vi "_testStepCfgEditor.vi"() -> ()   [LabVIEW 2010]
panel:
  in  "Generate testStepCfg.ini":bool
  out "View row details":string[](array[string])
  in  "Library function":string(tree)="library function"
  in  "Test Step CFG EDIT":string[][](table)
  out "error out":errorcluster
  in  "error in":errorcluster
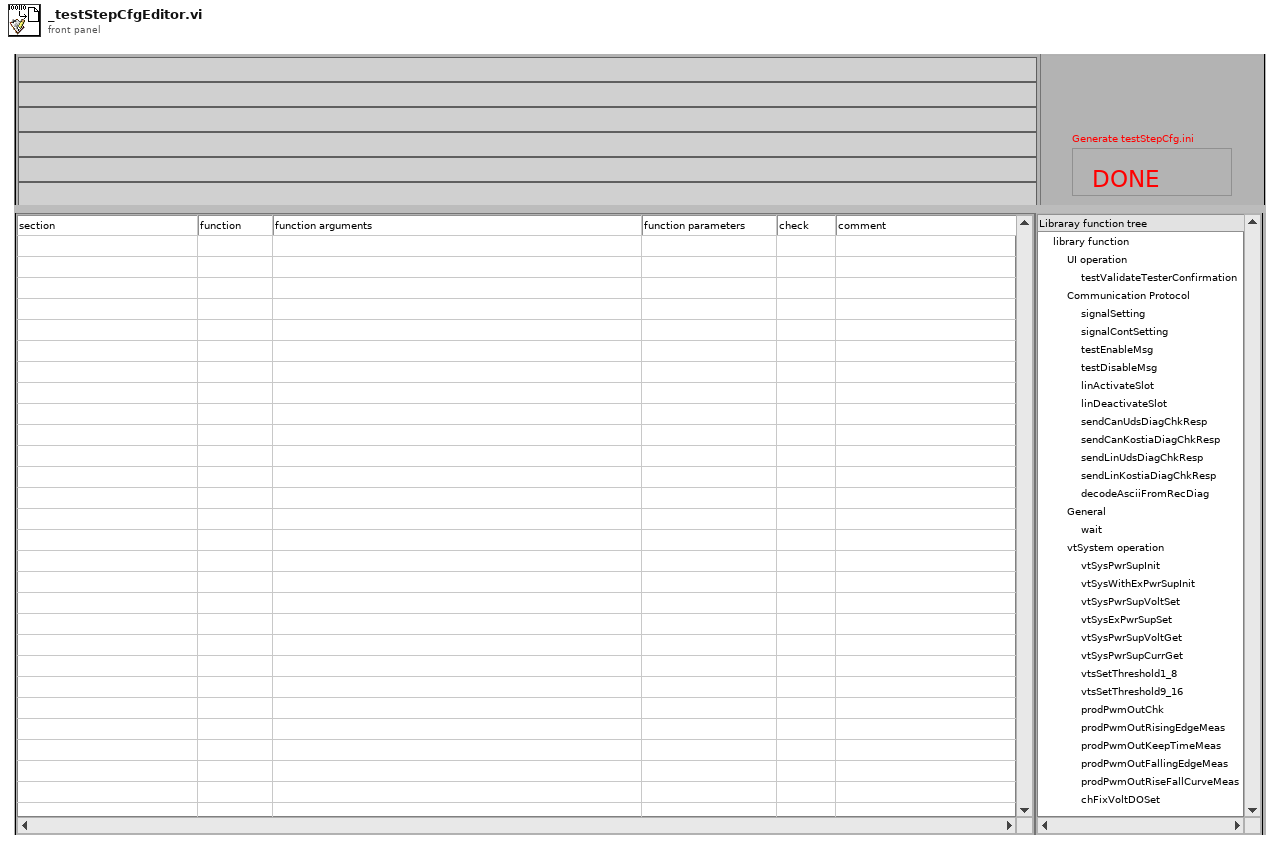
[diagram p1: front panel]
types:
  T1 = typedef "LVRowAndColumnTypeDef.ctl" = cluster{"Row":i32, "Column":i32}
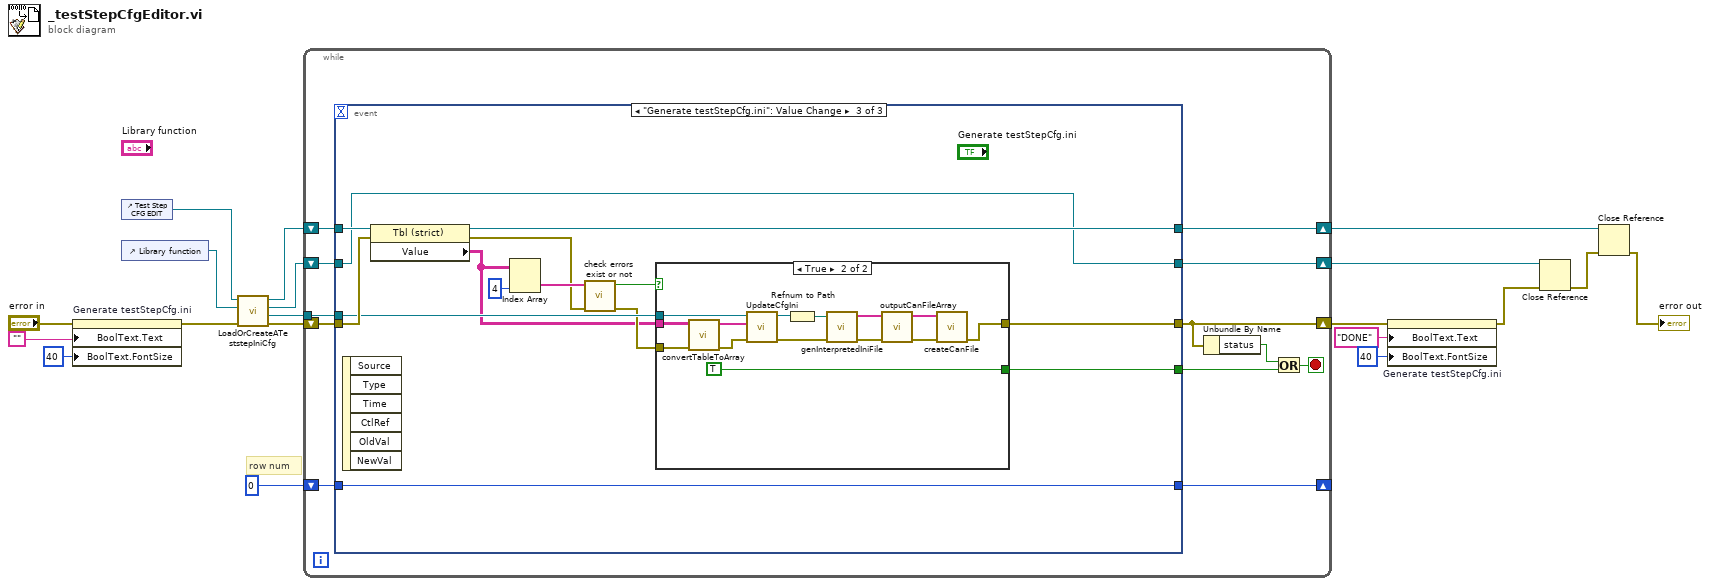
[diagram p0: block diagram]
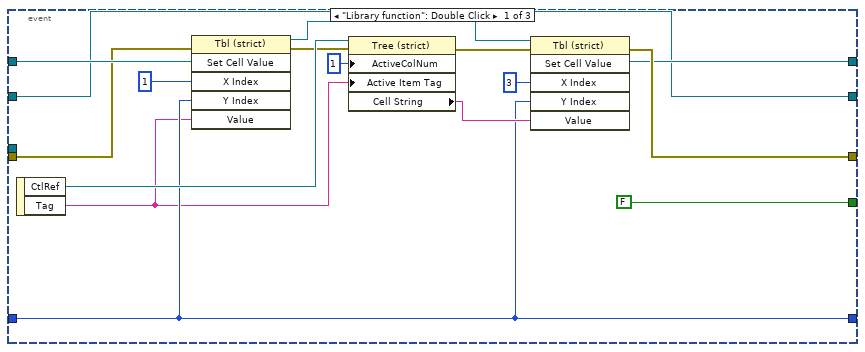
[diagram p2: hidden frame]
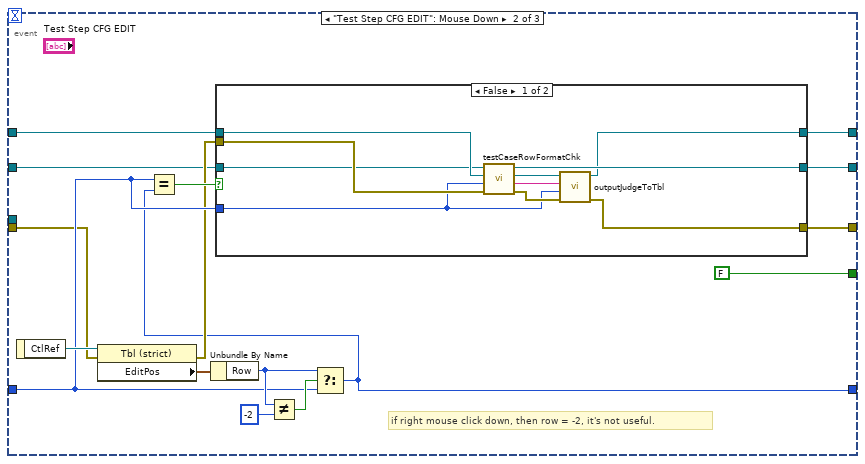
[diagram p3: hidden frame]
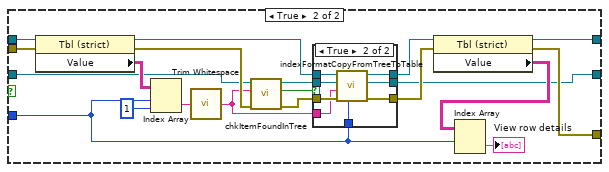
[diagram p4: hidden frame]
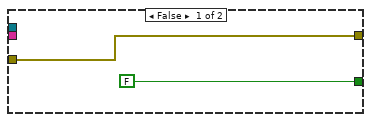
[diagram p6: hidden frame]
diagram:
  # "row num"
  n1 = property on="Generate testStepCfg.ini" class="Bool"(error in="error in", "BoolText.Text"="", "BoolText.FontSize"=u32 40 ("Boolean Text.Font:Size")) -> (error out=w8:errorcluster)  [unwired: 1 in, 1 out]
  n2 = control-ref of="Test Step CFG EDIT"() -> (w18:refnum<vi>)
  n3 = control-ref of="Library function"() -> (w19:refnum<vi>)
  n4 = call "LoadOrCreateATeststepIniCfg.vi"("error in"=w8, "Tree Refnum"=w19, "Tbl Refnum in"=w18) -> ("error out"=w12:errorcluster, "cfg file refnum out"=w16:refnum<file>, "Tree Refnum out"=w11:refnum<vi>, "Tbl Refnum out"=w13:refnum<vi>)  [unwired: 5 in]
  n5 = while {
    shift-right: [w28] -> w4
    shift-left: w12 -> [w31]
    shift-right: [w24] -> _
    shift-left: 0 ("Row") -> [w25]
    shift-right: [w23] -> w15
    shift-left: w13 -> [w26]
    tunnel: w16 -> [w22]
    shift-right: [w20] -> w10
    shift-left: w11 -> [w21]
    stop <- w29 stop-if-true
    n6 = event shown="[2] \"Generate testStepCfg.ini \": Value Change" {
      selector: _ -> [_ _ _]
      dyn-events: _ -> [_ _ _]
      timeout: _ -> [_ _ _]
      tunnel: w31 -> [w46 w53 w114]
      tunnel: [w37 w58 w115] -> w28
      tunnel: [FALSE ("stop") FALSE ("stop") w118] -> w30
      tunnel: w26 -> [w47 w48 w116]
      tunnel: w25 -> [w35 w55 w117]
      tunnel: [w35 w49 w117] -> w24
      tunnel: [w34 w56 w109] -> w23
      tunnel: w22 -> [_ _ w113]
      tunnel: w21 -> [w33 w51 w105]
      tunnel: [w33 w50 w105] -> w20
      event "Library function": Double Click {
        n7 = event-data() -> ("CtlRef"=w44:refnum<vi>, "Tag"=w32:string)  [unwired: 1 in]
        n8 = invoke class="Tbl (strict)" method="Set Cell Value"(reference=w47, error in=w46, "X Index"=u32 1 ("Y Index"), "Y Index"=w35, "Value"=w32) -> (reference out=w38:refnum<vi>, error out=w39:errorcluster)  [unwired: 1 in, 4 out]
        n9 = property class="Tree (strict)"(reference=w44, error in=w39, "ActiveColNum"=1 ("Active Cell:Active Column Number"), "Active Item Tag"=w32) -> (error out=w42:errorcluster, "Cell String"=w41:string)  [unwired: 1 out]
        n10 = invoke class="Tbl (strict)" method="Set Cell Value"(reference=w38, error in=w42, "X Index"=u32 3, "Y Index"=w35, "Value"=w41) -> (reference out=w34:refnum<vi>, error out=w37:errorcluster)  [unwired: 1 in, 4 out]
      }
      event "Test Step CFG EDIT": Mouse Down {
        # "if right mouse click down, then row = -2, it's not useful."
        n11 = event-data() -> ("CtlRef"=w63:refnum<vi>)  [unwired: 1 in]
        n12 = property class="Tbl (strict)"(reference=w63, error in=w53) -> (error out=w52:errorcluster, "EditPos"=w62:T1)  [unwired: 1 out]
        n13 = Unbundle By Name(w62) -> ("Row"=w59:i32)
        n14 = Not Equal?(x=w59, y=-2) -> (x != y?=w60:bool)
        n15 = Select(t=w59, s=w60, f=w55) -> (s? t:f=w49:i32)
        n16 = Equal?(x=w55, y=w49) -> (x = y?=w57:bool)
        n17 = case shown="False" w57 {
          tunnel: w55 -> [w67 w77]
          tunnel: w48 -> [w72 w91]
          tunnel: w52 -> [w73 w90]
          tunnel: [w64 w83] -> w58
          tunnel: [w65 w92] -> w56
          tunnel: w51 -> [w71 w85]
          tunnel: [w70 w74] -> w50
          frame False {
            n18 = call "testCaseRowFormatChk.vi"("error in"=w73, "Row number"=w67, "Tbl Refnum in"=w72, "Tree Refnum in"=w71) -> ("error out"=w68:errorcluster, "Check result"=w69:string, "Tbl Refnum out"=w66:refnum<vi>, "Tree Refnum out"=w70:refnum<vi>)  [unwired: 4 in]
            n19 = call "outputJudgeToTbl.vi"("error in"=w68, "rowNum"=w67, "judgeRes"=w69, "Tbl Refnum in"=w66) -> ("error out"=w64:errorcluster, "Tbl Refnum Out"=w65:refnum<vi>)  [unwired: 6 in]
          }
          frame True {
            n20 = property class="Tbl (strict)"(reference=w91, error in=w90) -> (reference out=w79:refnum<vi>, error out=w86:errorcluster, "Value"=w89:string[][])
            n21 = Index Array(array=w89, index (row)=w77, index (col)=1 ("disabled index (col)")) -> (element=w87:string)
            n22 = call <vilib>:"Trim Whitespace.vi"("string"=w87) -> ("trimmed string"=w78:string)  [unwired: 1 in]
            n23 = call "chkItemFoundInTree.vi"("error in"=w86, "searchItem"=w78, "Tree Refnum in"=w85) -> ("error out"=w82:errorcluster, "FoundInTree?"=w81:bool, "Tree Refnum out"=w80:refnum<vi>)  [unwired: 6 in]
            n24 = case shown="True" w81 {
              tunnel: [w96 w104] -> w76
              tunnel: [w94 w103] -> w75
              tunnel: w77 -> [_ w102]
              tunnel: [w95 w101] -> w74
              tunnel: w80 -> [w95 w100]
              tunnel: w82 -> [w94 w99]
              tunnel: w79 -> [w96 w98]
              tunnel: w78 -> [_ w97]
              frame False {
              }
              frame True {
                n25 = call "indexFormatCopyFromTreeToTable.vi"("rowNum"=w102, "error in"=w99, "searchItem"=w97, "Tree Refnum In"=w100, "Tbl Refnum in"=w98) -> ("error out"=w103:errorcluster, "Tree Refnum Out"=w101:refnum<vi>, "Tbl Refnum Out"=w104:refnum<vi>)  [unwired: 4 in]
              }
            }
            n26 = property class="Tbl (strict)"(reference=w76, error in=w75) -> (reference out=w92:refnum<vi>, error out=w83:errorcluster, "Value"=w84:string[][])
            n27 = Index Array(array=w84, index (row)=w77) -> (element=→"View row details":string[])  [unwired: 1 in]
          }
        }
      }
      event "Generate testStepCfg.ini": Value Change {
        n28 = event-data() -> ()  [unwired: 1 in, 6 out]
        n29 = property class="Tbl (strict)"(reference=w116, error in=w114) -> (reference out=w109:refnum<vi>, error out=w110:errorcluster, "Value"=w106:string[][])
        n30 = Index Array(array=w106, index (col)=4 ("disabled index (col)")) -> (element=w111:string[])  [unwired: 1 in]
        n31 = call "check errors exist or not.vi"("error in"=w110, "judge column"=w111) -> ("error out"=w108:errorcluster, "Go on?"=w107:bool)  [unwired: 8 in]
        n32 = case shown="True" w107 {
          tunnel: [FALSE ("stop") TRUE ("stop")] -> w118
          tunnel: [w119 w130] -> w115
          tunnel: w113 -> [_ w131]
          tunnel: w108 -> [w119 w133]
          tunnel: w106 -> [_ w127]
          frame False {
          }
          frame True {
            n33 = call "convertTableToArray.vi"("error in"=w133, "tbl"=w127) -> ("error out"=w132:errorcluster, "contArr"=w129:string[])  [unwired: 8 in]
            n34 = call "UpdateCfgIni.vi"("error in"=w132, "contentArray"=w129, "iniCfgRefnumIn"=w131) -> ("error out"=w125:errorcluster, "iniCfgRefnumOut"=w121:refnum<file>)  [unwired: 7 in]
            n35 = Refnum to Path(1:w121) -> (0:w122:path)
            n36 = call "genInterpretedIniFile.vi"("error in"=w125, "configuration file path"=w122) -> ("error out"=w124:errorcluster, "interpretedIniFileContentArray"=w123:string[])  [unwired: 8 in]
            n37 = call "outputCanFileArray.vi"("error in"=w124, "interpretedIniFileContentArray"=w123) -> ("error out"=w128:errorcluster, "testCaseInCanFileArr"=w126:string[])  [unwired: 8 in]
            n38 = call "createCanFile.vi"("error in"=w128, "contentArray"=w126) -> ("error out"=w130:errorcluster)  [unwired: 9 in]
          }
        }
      }
    }
    n39 = Unbundle By Name(w28) -> ("status"=w27:bool)
    n40 = Or(x=w27, y=w30) -> (x .or. y?=w29:bool)
  }
  n41 = property on="Generate testStepCfg.ini" class="Bool"(error in=w4, "BoolText.Text"="DONE" ("Boolean Text.Text"), "BoolText.FontSize"=u32 40 ("Boolean Text.Font:Size")) -> (error out=w1:errorcluster)  [unwired: 1 in, 1 out]
  n42 = Close Reference(reference=w10, error in (no error)=w1) -> (error out=w9:errorcluster)
  n43 = Close Reference(reference=w15, error in (no error)=w9) -> (error out=→"error out":errorcluster)
